vi "Experiment_GUIDE_WAVELENGTH.vi"() -> ()   [LabVIEW 2009]
uses:
  <vilib>/imath/engines/lvmath2/RunTimeEngine/ErrorHandling/NIMS_Finalize Error.vi
  <vilib>/imath/engines/lvmath2/RunTimeEngine/Parser/MC_Version.vi
  <vilib>/imath/engines/lvmath2/RunTimeEngine/Managers/WorkSpace/UID Generator.vi
  <vilib>/imath/engines/lvmath2/RunTimeEngine/NodeEndStatement/NIMS_NodeEndStatement_Output.vi
  <instcachedir>/0/NIMS_NodeEndStatement_Output_B70DDD75627E4997AAE11E9955EDAA25.lvgen/NIMS_NodeEndStatement_Output_B70DDD75627E4997AAE11E9955EDAA25_001.vi
  <vilib>/imath/engines/lvmath2/RunTimeEngine/Managers/SymbolTable/Clear UID.vi
  <vilib>/imath/engines/lvmath2/RunTimeEngine/LocalVariableDefStatement/MC_LocalVariableDefStatement_Display.vi
  <vilib>/imath/engines/lvmath2/RunTimeEngine/RunTimeType/NIMS_RunTimeType_From StrictType (excl LVString).vi
  <vilib>/imath/engines/lvmath2/RunTimeEngine/RangeToken/NIMS_Range.vi
  <instcachedir>/0/NIMS_Range_6D647EC16A744C98B5DE1D649A2D648D.lvgen/NIMS_Range_6D647EC16A744C98B5DE1D649A2D648D_001.vi
  <vilib>/imath/engines/lvmath/Functions/Error Handling/error.ctl
  <vilib>/imath/engines/lvmath/Functions/Error Handling/MergeErrorsWrapper.vi
  <vilib>/imath/engines/lvmath2/RunTimeEngine/VariableToken/NIMS_VariableToken_CondDefined.vi
  <instcachedir>/0/NIMS_VariableToken_CondDefined_5641E79000FB4D628475532441475385.lvgen/NIMS_VariableToken_CondDefined_5641E79000FB4D628475532441475385_002.vi
  <vilib>/imath/engines/lvmath/Functions/Error Handling/MC_Mask_Errors.vi
  <vilib>/imath/engines/lvmath2/RunTimeEngine/BuiltInFunctions/rem/NIMS_rem_no checks.vi
  <instcachedir>/0/NIMS_rem_no checks_4CC9B305AB7E42EF90AFC4973FB32F8D.lvgen/NIMS_rem_no checks_4CC9B305AB7E42EF90AFC4973FB32F8D_000.vi
  <vilib>/imath/engines/lvmath2/RunTimeEngine/BuiltInFunctions/uint32/NIMS_uint32(real).vi
  <instcachedir>/0/NIMS_uint32(real)_FDC83D68D45943DDB8F3F934FF8A712F.lvgen/NIMS_uint32(real)_FDC83D68D45943DDB8F3F934FF8A712F_000.vi
  <vilib>/imath/engines/lvmath2/RunTimeEngine/BuiltInFunctions/double/NIMS_double.vi
  <instcachedir>/0/NIMS_double_2CE444F3CE4146B199A482FE12545E45.lvgen/NIMS_double_2CE444F3CE4146B199A482FE12545E45_000.vi
  <vilib>/imath/engines/lvmath2/RunTimeEngine/BuiltInFunctions/length/NIMS_length(GV).vi
  <instcachedir>/0/NIMS_length(GV)_7D6E94E728E145E68721C53861296D96.lvgen/NIMS_length(GV)_7D6E94E728E145E68721C53861296D96_000.vi
  <instcachedir>/0/NIMS_Range_6D647EC16A744C98B5DE1D649A2D648D.lvgen/NIMS_Range_6D647EC16A744C98B5DE1D649A2D648D_000.vi
  <vilib>/imathl/engines/lvmath/Functions/Error Handling/Create Error.vi
  <vilib>/imath/engines/lvmath2/RunTimeEngine/ReplaceToken/NIMS_Replace - V(S)=S.vi
  <instcachedir>/0/NIMS_Replace - V(S)=S_670A9E0533664C1D848C8E58B3321B6A.lvgen/NIMS_Replace - V(S)=S_670A9E0533664C1D848C8E58B3321B6A_001.vi
  <vilib>/imath/engines/lvmath2/RunTimeEngine/ReplaceToken/NIMS_Replace - Size Check _(_)=S.vi
  <instcachedir>/0/NIMS_Replace - Size Check _(_)=S_8596181D73404097BAB9CBB006194BB0.lvgen/NIMS_Replace - Size Check _(_)=S_8596181D73404097BAB9CBB006194BB0_002.vi
  <vilib>/imath/engines/lvmath2/RunTimeEngine/ReplaceToken/NIMS_Replace - Check Linear.vi
  <instcachedir>/0/NIMS_Replace - Check Linear_9243CBB174894FF6977027453DA6955E.lvgen/NIMS_Replace - Check Linear_9243CBB174894FF6977027453DA6955E_002.vi
  <vilib>/imath/engines/lvmath2/RunTimeEngine/VariableToken/NIMS_VariableToken_CondDefinedDefinedByReplace.vi
  <instcachedir>/0/NIMS_VariableToken_CondDefinedDefinedByReplace_D162CFFC24174562A9FEA619A91E1A56.lvgen/NIMS_VariableToken_CondDefinedDefinedByReplace_D162CFFC24174562A9FEA619A91E1A56_002.vi
  <vilib>/imath/engines/lvmath2/RunTimeEngine/CommandStatement/MC_CommandStatement_break.vi
  <vilib>/imath/engines/lvmath2/RunTimeEngine/ArithmeticOperatorToken/NIMS_ArithmeticOperator_times.vi
  <instcachedir>/0/NIMS_ArithmeticOperator_times_3987BC660D7947CD8628C10658A43225.lvgen/NIMS_ArithmeticOperator_times_3987BC660D7947CD8628C10658A43225_001.vi
  <instcachedir>/0/NIMS_NodeEndStatement_Output_B70DDD75627E4997AAE11E9955EDAA25.lvgen/NIMS_NodeEndStatement_Output_B70DDD75627E4997AAE11E9955EDAA25_000.vi
  <instcachedir>/0/NIMS_ArithmeticOperator_times_3987BC660D7947CD8628C10658A43225.lvgen/NIMS_ArithmeticOperator_times_3987BC660D7947CD8628C10658A43225_000.vi
  <vilib>/imath/engines/lvmath2/RunTimeEngine/VariableToken/Read/NIMS_Get Elements - RV(_) - Check.vi
  <instcachedir>/0/NIMS_Get Elements - RV(_) - Check_60F12861D0564803969A5D0D0D1716CD.lvgen/NIMS_Get Elements - RV(_) - Check_60F12861D0564803969A5D0D0D1716CD_001.vi
  <instcachedir>/0/NIMS_NodeEndStatement_Output_B70DDD75627E4997AAE11E9955EDAA25.lvgen/NIMS_NodeEndStatement_Output_B70DDD75627E4997AAE11E9955EDAA25_002.vi
  <instcachedir>/0/NIMS_VariableToken_CondDefined_5641E79000FB4D628475532441475385.lvgen/NIMS_VariableToken_CondDefined_5641E79000FB4D628475532441475385_001.vi
  <instcachedir>/0/NIMS_Replace - V(S)=S_670A9E0533664C1D848C8E58B3321B6A.lvgen/NIMS_Replace - V(S)=S_670A9E0533664C1D848C8E58B3321B6A_000.vi
  <instcachedir>/0/NIMS_Replace - Size Check _(_)=S_8596181D73404097BAB9CBB006194BB0.lvgen/NIMS_Replace - Size Check _(_)=S_8596181D73404097BAB9CBB006194BB0_001.vi
  <instcachedir>/0/NIMS_Replace - Check Linear_9243CBB174894FF6977027453DA6955E.lvgen/NIMS_Replace - Check Linear_9243CBB174894FF6977027453DA6955E_001.vi
  <instcachedir>/0/NIMS_VariableToken_CondDefinedDefinedByReplace_D162CFFC24174562A9FEA619A91E1A56.lvgen/NIMS_VariableToken_CondDefinedDefinedByReplace_D162CFFC24174562A9FEA619A91E1A56_001.vi
  <vilib>/imath/engines/lvmath2/RunTimeEngine/BuiltInFunctions/abs/NIMS_abs(signed).vi
  <instcachedir>/0/NIMS_abs(signed)_C4FCB8E6058B49B797C7C8D53CA5F6EC.lvgen/NIMS_abs(signed)_C4FCB8E6058B49B797C7C8D53CA5F6EC_000.vi
  <instcachedir>/0/NIMS_NodeEndStatement_Output_B70DDD75627E4997AAE11E9955EDAA25.lvgen/NIMS_NodeEndStatement_Output_B70DDD75627E4997AAE11E9955EDAA25_003.vi
  <vilib>/imath/engines/lvmath2/RunTimeEngine/Managers/SymbolTable/NIMS_WorkSpace.lvlib
panel:
  in  "?":T1(tab)
  in  "?":dbl(slide) scale=0.1..0.5
  in  "?":enum32{"IMPEDANCE OF HORN ANTENNA"}(tab)
  in  "Reactance of Horn":dbl(slide) scale=0.0..500.0
  in  "Resistance of Horn":dbl(slide) scale=0.0..500.0
  in  "?":enum32{"SLOTTED LINE"}(tab)
  out "?":dbl[](graph)
  out "Characteristic Impedance":dbl
  in  "Slide":dbl(slide) scale=0.0..0.4
  out "Voltage":dbl
  out "Distance(Meter)":dbl
  in  "First Freespace Minima":bool
  in  "Second Freespace Minima":bool
  in  "First Wave-guideMinima":bool
  out "?":dbl
  out "?":dbl
  out "?":dbl
  in  "Second Wave-guide Minima":bool
  out "?":dbl
  out "?":errorcluster
  out "?":dbl
  in  "Width of the Wave-guide":bool
  in  "HELP FOR SLOTTED LINE":bool
  out "error out":errorcluster
  in  "?":enum32{"ATTENUATOR"}(tab)
  out "?":dbl[](graph)
  out "?":errorcluster
  in  "Set the value of attenuation in dB":dbl(slide) scale=0.0..100.0
  in  "HELP FOR ATTENUATOR":bool
  out "error out":errorcluster
  in  "?":enum32{"ISOLATOR"}(tab)
  out "?":dbl[](graph)
  out "?":errorcluster
  in  "?":bool
  in  "HELP FOR ISOLATOR":bool
  out "error out":errorcluster
  in  "?":enum32{"MODULATOR"}(tab)
  out "?":dbl[](graph)
  out "?":errorcluster
  in  "Modulating Frequency(KHz)":dbl(slide) scale=0.5..1.5
  in  "HELP FOR MODULATOR":bool
  out "error out":errorcluster
  in  "?":enum32{"SOURCE"}(tab)
  out "?":dbl[](graph)
  out "?":errorcluster
  in  "Voltage":dbl(knob) scale=0.0..20.0 scale format="%#_10g"
  in  "Frequency of carrier wave(GHz)":dbl(slide) scale=8.0..15.0
  in  "HELP FOR SOURCE":bool
  out "error out":errorcluster
  # "VSWR Meter"
  # "Source"
  # "Variable Attenuator"
  # "Slotted Line"
  # "Metal plate"
  # "Horn Antenna"
  # "Coaxial to rectangular adapter"
  # "Isolator"
  # "Connecting waveguide"
  # "Connecting waveguide"
  # "Connecting waveguide"
  # "Backward Direction"
  # "Forward direction"
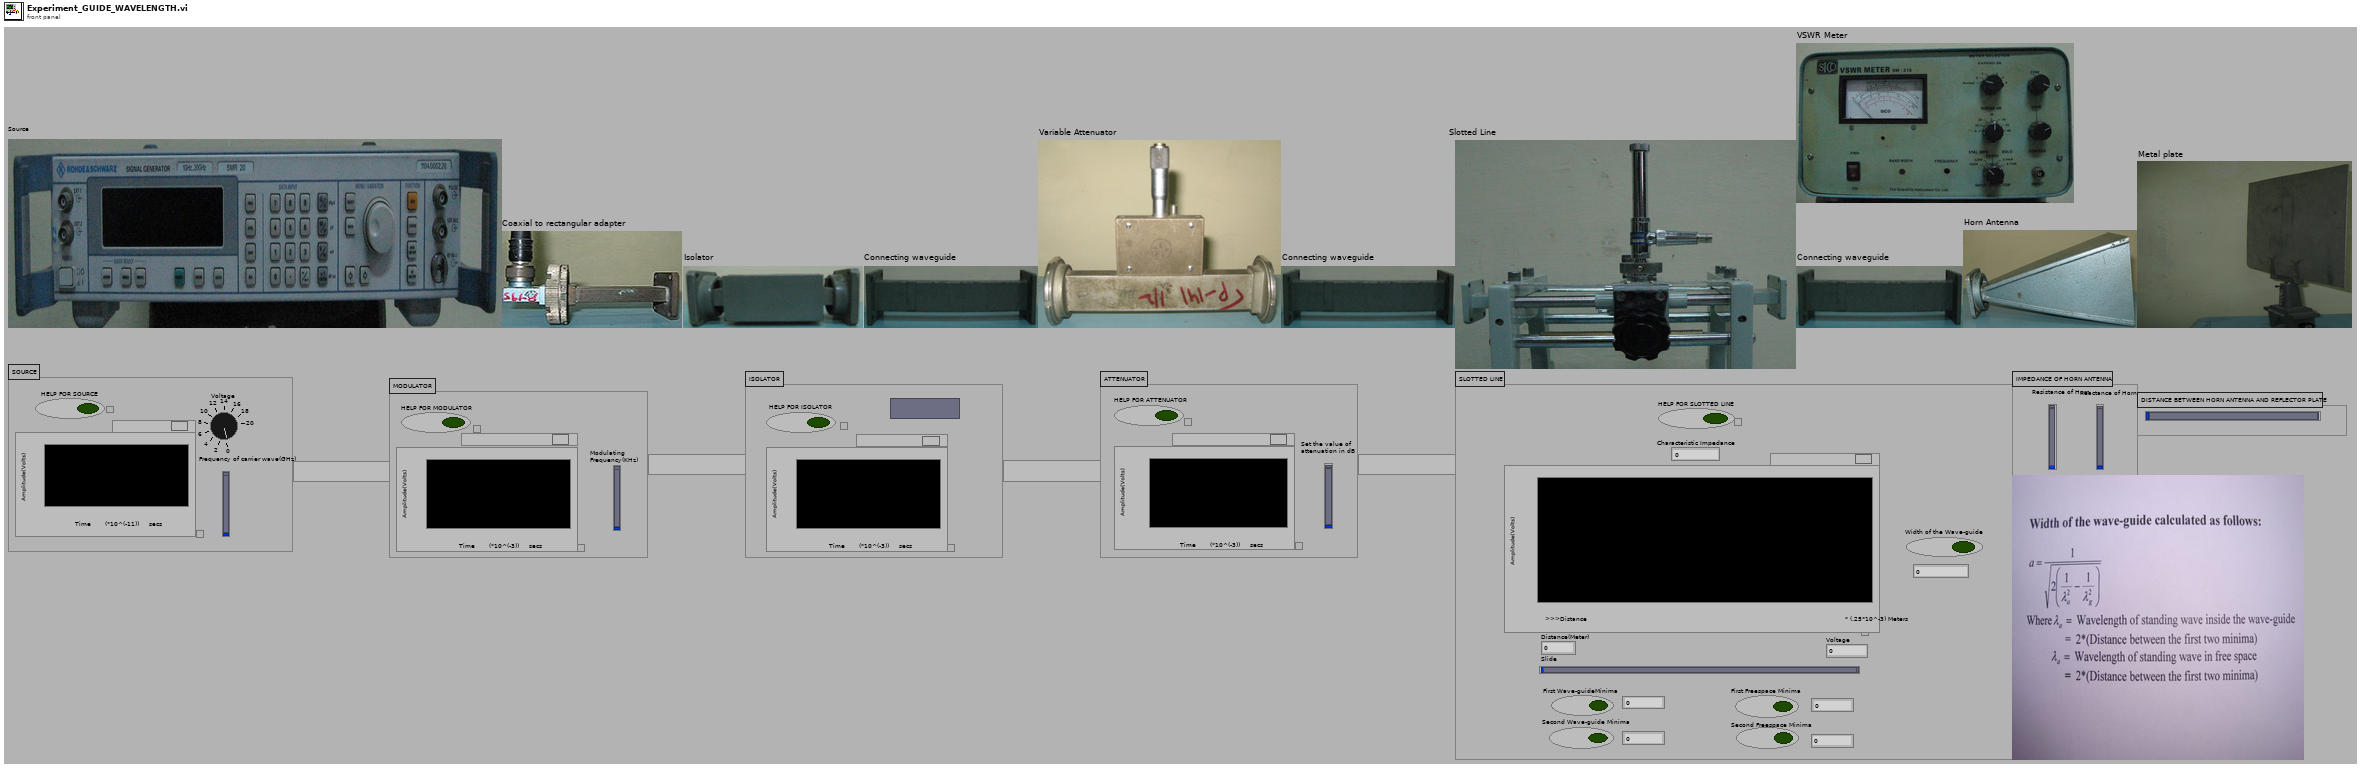
[diagram p1: front panel]
types:
  T1 = enum32{"DISTANCE BETWEEN HORN ANTENNA AND REFLECTOR PLATE"}
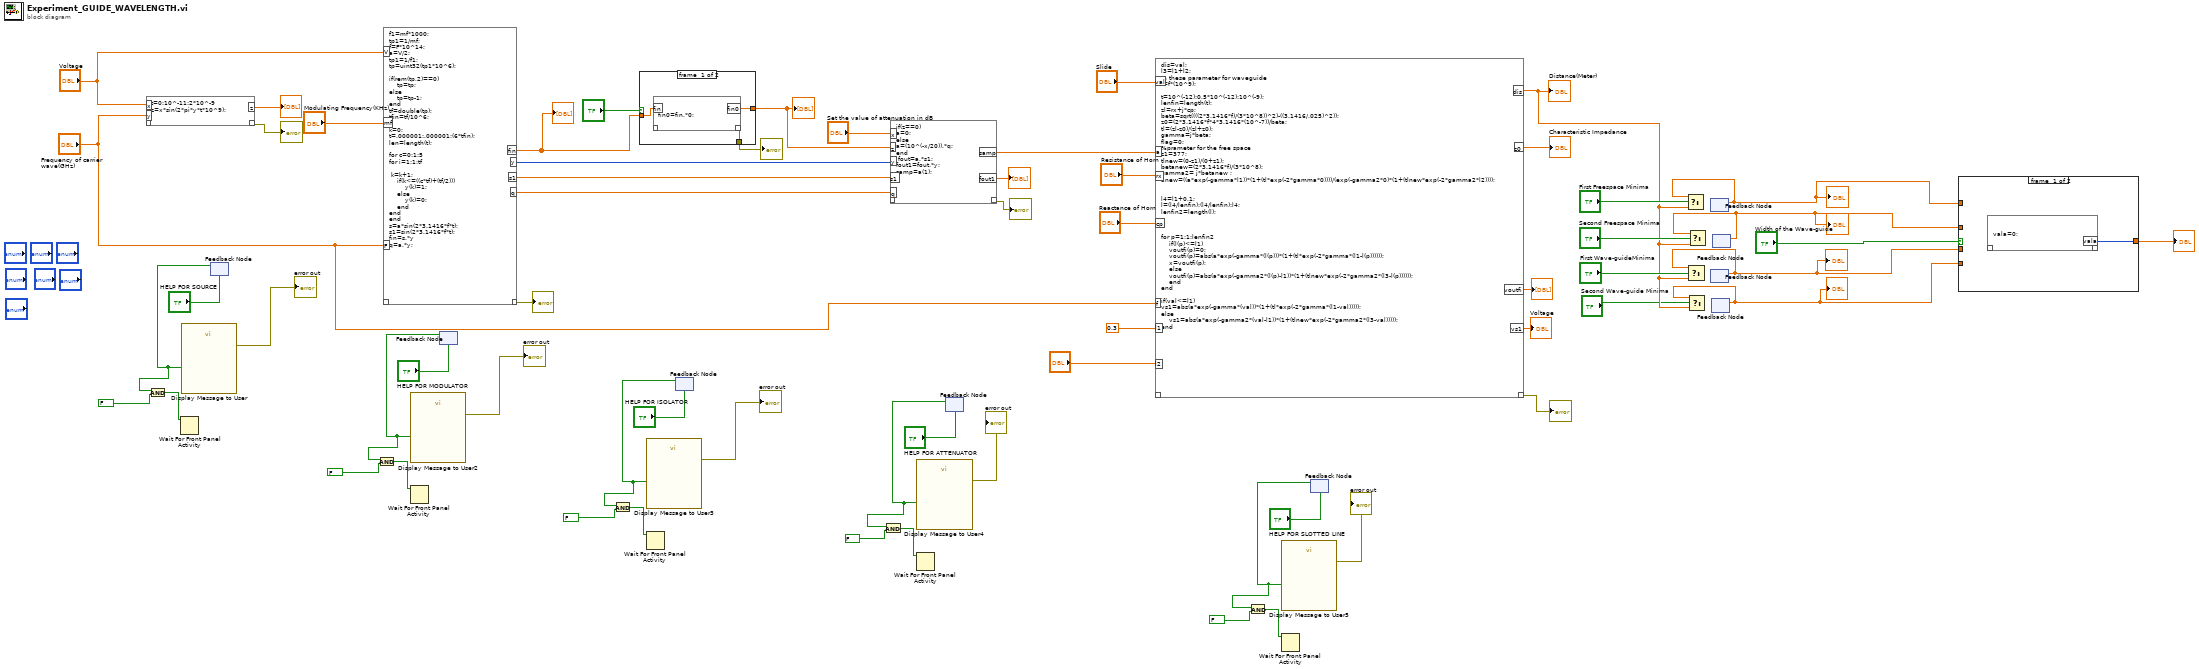
[diagram p0: block diagram]
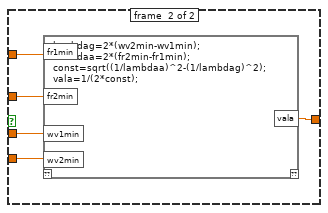
[diagram p2: hidden frame]
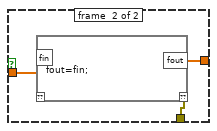
[diagram p3: hidden frame]
diagram:
  n1 = mathscript code="t=0:10^-11:2*10^-9\nz=x*sin(2*pi*y*t*10^9);"("x"="Voltage", "y"="Frequency of carrier wave(GHz)") -> ("??"=→"?":errorcluster, "z"=→"?":dbl[])  [unwired: 1 in]
  n2 = feedback #1("HELP FOR SOURCE") -> (w67:bool)
  n3 = And(x=w67, y=FALSE) -> (x .and. y?=w65:bool)
  n4 = Wait For Front Panel Activity(3:w65) -> ()  [unwired: 3 out]
  n5 = call "Display Message to User"("Enable"=w67) -> ("error out"=→"error out":errorcluster, "CLOSE"=w69:bool)  [unwired: 2 in, 7 out]
  n6 = mathscript code="f1=mf*1000;\ntp1=1/mf;\nf=F*10^14;\na=V/2;\ntp1=1/f1;\ntp=uint32(tp1*10^6);\n\nif(rem(tp,2)==0)\n    tp=tp;\nelse\n    tp=tp-1;\nend\ntf=double(tp);\ntfin=tf/10^6;\n\nk=0;\nt=.000001:.000001:(6*tfin);\nlen=length(t);\n\nfor c=0:1:5\nfor i=1:1:tf\n  \n k=k+1;\n    if(k<=((c*tf)+(tf/2)))\n        y(k)=1;\n    else\n        y(k)=0;\n    end\nend\nend\ns=a*sin(2*3.1416*f*t);\ns1=sin(2*3.1416*f*t);\nfin=s.*y\nq=a.*y;"("V"="Voltage", "mf"="Modulating Frequency(KHz)", "F"="Frequency of carrier wave(GHz)") -> ("??"=→"?":errorcluster, "fin"=w36:dbl[], "y"=w33:i32[], "s1"=w32:dbl[], "q"=w31:dbl[])  [unwired: 1 in]
  "?" <- w36
  n7 = feedback #2("HELP FOR MODULATOR") -> (w61:bool)
  n8 = And(x=w61, y=FALSE) -> (x .and. y?=w59:bool)
  n9 = Wait For Front Panel Activity(3:w59) -> ()  [unwired: 3 out]
  n10 = call "Display Message to User2"("Enable"=w61) -> ("error out"=→"error out":errorcluster, "CLOSE"=w63:bool)  [unwired: 2 in, 7 out]
  n11 = case shown="False" "?" {
    tunnel: [w73 w94] -> w2
    tunnel: w36 -> [w74 w95]
    tunnel: [w72 w93] -> w1
    frame #0 {
      n12 = mathscript code="fin0=fin.*0;"("fin"=w74) -> ("??"=w72:errorcluster, "fin0"=w73:dbl[])  [unwired: 1 in]
    }
    frame #1 {
      n13 = mathscript code="fout=fin;"("fin"=w95) -> ("??"=w93:errorcluster, "fout"=w94:dbl[])  [unwired: 1 in]
    }
  }
  "?" <- w2
  "?" <- w1
  n14 = feedback #3("HELP FOR ISOLATOR") -> (w55:bool)
  n15 = And(x=w55, y=FALSE) -> (x .and. y?=w53:bool)
  n16 = Wait For Front Panel Activity(3:w53) -> ()  [unwired: 3 out]
  n17 = call "Display Message to User3"("Enable"=w55) -> ("error out"=→"error out":errorcluster, "CLOSE"=w57:bool)  [unwired: 2 in, 7 out]
  n18 = mathscript code="if(z==0)\na=0; \nelse\na=(10^(-x/20)).*q;\nend\n fout=a.*s1;\nfout1=fout.*y;\nsamp=a(1);"("x"="Set the value of attenuation in dB", "z"=w2, "y"=w33, "s1"=w32, "q"=w31) -> ("??"=→"?":errorcluster, "samp"=w27:dbl, "fout1"=→"?":dbl[])  [unwired: 1 in]
  n19 = feedback #4("HELP FOR ATTENUATOR") -> (w49:bool)
  n20 = And(x=w49, y=FALSE) -> (x .and. y?=w47:bool)
  n21 = Wait For Front Panel Activity(3:w47) -> ()  [unwired: 3 out]
  n22 = call "Display Message to User4"("Enable"=w49) -> ("error out"=→"error out":errorcluster, "CLOSE"=w51:bool)  [unwired: 2 in, 7 out]
  n23 = mathscript code="dis=val;\nl3=l1+l2;\n% these parameter for waveguide\nf=f*(10^9);\n\nt=10^(-12):0.5*10^(-12):10^(-9);\nlenfin=length(t);\nzl=rx+j*cp;\nbeta=sqrt((((2*3.1416*f)/(3*10^8))^2)-((3.1416/.025)^2));\nz0=(2*3.1416*f*4*3.1416*(10^-7))/beta;\ntl=(zl-z0)/(zl+z0);\ngamma=j*beta;\nflag=0;\n%prameter for the free space\nz1=377;\ntlnew=(0-z1)/(0+z1);\nbetanew=(2*3.1416*f)/(3*10^8);\ngamma2= j*betanew ;\nanew=((a*exp(-gamma*l1))*(1+(tl*exp(-2*gamma*0))))/(exp(-gamma2*0)*(1+(tlnew*exp(-2*gamma2*l2))));\n\n\nl4=l1+0.1;\nl=(l4/lenfin):(l4/lenfin):l4;\nlenfin2=length(l);\n\n\n\nfor p=1:1:lenfin2\n    if(l(p)<=l1)\n    voutfi(p)=0;\n    voutfi(p)=abs(a*exp(-gamma*(l(p)))*(1+(tl*exp(-2*gamma*(l1-l(p))))));\n    x=voutfi(p);\n    else\n    voutfi(p)=abs(a*exp(-gamma2*(l(p)-l1))*(1+(tlnew*exp(-2*gamma2*(l3-l(p))))));\n    end\nend\n\nif(val<=l1)\nvs1=abs(a*exp(-gamma*(val))*(1+(tl*exp(-2*gamma*(l1-val)))));\nelse\n    vs1=abs(a*exp(-gamma2*(val-l1))*(1+(tlnew*exp(-2*gamma2*(l3-val)))));\nend"("val"="Slide", "a"=w27, "rx"="Resistance of Horn", "cp"="Reactance of Horn", "f"="Frequency of carrier wave(GHz)", "l1"=0.3 ("Real"), "l2"="?") -> ("??"=→"?":errorcluster, "dis"=w5:dbl, "z0"=→"Characteristic Impedance":cdb, "voutfi"=→"?":dbl[], "vs1"=→"Voltage":dbl)  [unwired: 1 in]
  "Distance(Meter)" <- w5
  n24 = feedback #5("HELP FOR SLOTTED LINE") -> (w43:bool)
  n25 = And(x=w43, y=FALSE) -> (x .and. y?=w41:bool)
  n26 = Wait For Front Panel Activity(3:w41) -> ()  [unwired: 3 out]
  n27 = call "Display Message to User5"("Enable"=w43) -> ("error out"=→"error out":errorcluster, "CLOSE"=w45:bool)  [unwired: 2 in, 7 out]
  n28 = feedback #6() -> (w13:dbl)  [unwired: 1 in]
  "?" <- w13
  n29 = Select(t=w13, s="First Freespace Minima", f=w5) -> (s? t:f=w15:dbl)
  n30 = feedback #7() -> (w7:dbl)  [unwired: 1 in]
  "?" <- w7
  n31 = Select(t=w7, s="First Wave-guideMinima", f=w5) -> (s? t:f=w9:dbl)
  n32 = feedback #8() -> (w3:dbl)  [unwired: 1 in]
  "?" <- w3
  n33 = Select(t=w3, s="Second Wave-guide Minima", f=w5) -> (s? t:f=w6:dbl)
  n34 = feedback #9() -> (w10:dbl)  [unwired: 1 in]
  "?" <- w10
  n35 = Select(t=w10, s="Second Freespace Minima", f=w5) -> (s? t:f=w12:dbl)
  n36 = case shown="True" "Width of the Wave-guide" {
    tunnel: [w112 w127] -> w17
    tunnel: w13 -> [_ w131]
    tunnel: w10 -> [_ w130]
    tunnel: w7 -> [_ w129]
    tunnel: w3 -> [_ w128]
    frame #0 {
      n37 = mathscript code="vala=0;"() -> ("vala"=w112:i32)  [unwired: 1 in, 1 out]
    }
    frame #1 {
      n38 = mathscript code="lambdag=2*(wv2min-wv1min);\nlambdaa=2*(fr2min-fr1min);\nconst=sqrt((1/lambdaa)^2-(1/lambdag)^2);\nvala=1/(2*const);"("fr1min"=w131, "fr2min"=w130, "wv1min"=w129, "wv2min"=w128) -> ("vala"=w127:cdb)  [unwired: 1 in, 1 out]
    }
  }
  "?" <- w17
